vi "s.vi"() -> ()   [LabVIEW 2013] (continued)
          n587 = local read "String"() -> (w1170:string)
          n588 = Equal?(x=w1170, y=w1175) -> (x = y?=w1172:bool)
          n589 = case shown="False" w1172 {
            tunnel: w1171 -> [w1180 _]
            tunnel: [w1179 w1208] -> w1169
            tunnel: w1168 -> [w1179 _]
            frame False {
              n590 = case shown="True" w1179 {
                tunnel: w1180 -> [_ w1185]
                frame False {
                }
                frame True {
                  n591 = case shown="1" "flag 8" {
                    tunnel: [w1206 w1207] -> w1189
                    tunnel: [w1206 w1207] -> w1193
                    frame 0, Default {
                      w1206 = "Admin"
                    }
                    frame 1 {
                      w1207 = "User"
                    }
                  }
                  n592 = Concatenate Strings("String", "-" ("string"), "String", ":" ("string"), w1189) -> (w1197:string)
                  n593 = local read "Numeric"() -> (w1196:dbl)
                  n594 = Open/Create/Replace File(file path (use dialog)=path "C:/Users/kiat/Desktop/password.txt" ("file (use dialog)")) -> (refnum out=w1183:refnum<file>)  [unwired: 5 in, 2 out]
                  n595 = local read "Table Control"() -> (w1194:string[][])
                  n596 = Build Array("String", "String", w1193) -> (w1190:string[])
                  n597 = case shown="0, Default" w1196 {
                    tunnel: [w1199 w1205] -> w1182
                    tunnel: w1185 -> [w1201 w1204]
                    tunnel: w1197 -> [w1200 w1202]
                    frame 0, Default {
                      n598 = Concatenate Strings(w1201, w1200) -> (w1199:string)
                      n599 = local write "Numeric"(0.0) -> ()
                    }
                    frame 1 {
                      n600 = Concatenate Strings(w1204, "\n", w1202) -> (w1205:string)
                    }
                  }
                  n601 = Write to Text File(file (use dialog)=w1183, text=w1182) -> (refnum out=w1184:refnum<file>)  [unwired: 2 in, 2 out]
                  n602 = Insert Into Array(array=w1194, new element=w1190) -> (w1195:string[][])  [unwired: 2 in]
                  n603 = local write "Table Control"(w1195) -> ()
                  n604 = Close File(refnum=w1184) -> ()  [unwired: 1 in, 2 out]
                }
              }
            }
            frame True {
              n605 = call "Display Message to User2"("Message"="Please choose another name") -> ("OK"=w1208:bool)  [unwired: 9 in, 1 out]
            }
          }
        }
        n606 = Close File(refnum=w1167) -> ()  [unwired: 1 in, 2 out]
      }
      event "edit": Value Change {
        n607 = event-data() -> ()  [unwired: 1 in, 6 out]
        n608 = property on="Table Control" class="Tbl (strict)"() -> ("Value"=w1433:string[][])  [unwired: 2 in, 2 out]
        n609 = local read "String"() -> (w1441:string)
        n610 = Read from Text File(file (use dialog)=w1440) -> (refnum out=w1454:refnum<file>, text=w1436:string, error out=w1460:errorcluster)  [unwired: 3 in, 1 out]
        n611 = Decimal String To Number(string=w1441) -> (number=w1434:i32)  [unwired: 2 in, 1 out]
        n612 = local read "Table Control"() -> (w1447:string[][])
        n613 = Array Size(array=w1433) -> (size(s)=w1443:i32[])
        n614 = local read "String"() -> (w1444:string)
        n615 = Add(x=1, y=w1434) -> (x+y=w1435:i32)
        n616 = Close File(refnum=w1454, error in=w1460) -> (path=w1451:path, error out=w1450:errorcluster)
        n617 = Index Array(array=w1443) -> (element=w1442:i32)  [unwired: 1 in]
        n618 = Decimal String To Number(string=w1444) -> (number=w1438:i32)  [unwired: 2 in, 1 out]
        n619 = Greater Or Equal?(x=w1435, y=w1442) -> (x >= y?=w1432:bool)
        n620 = case shown="True" w1432 {
          frame False {
          }
          frame True {
            n621 = local write "Table Control"(string[][] [] ("Table Control")) -> ()
            n622 = Read from Text File(file (use dialog)=path "C:/Users/kiat/Desktop/password.txt") -> (text=w1463:string)  [unwired: 3 in, 3 out]
            n623 = while {
              border: w1463 -> [_]
              stop <- w1473 stop-if-true
              n624 = feedback #2() -> (w1477:string)
              n625 = xnode "Match Regular Expression"("input string"=w1477, "regular expression"="\n") -> ("before match"=w1476:string, "after match"=w1475:string)  [unwired: 4 in, 3 out]
              n626 = feedback-in #2(w1475) -> ()
              n627 = xnode "Match Regular Expression"("input string"=w1476, "regular expression"="-") -> ("before match"=w1472:string, "after match"=w1471:string)  [unwired: 4 in, 3 out]
              n628 = Equal?(x=w1475, y="") -> (x = y?=w1473:bool)
              n629 = xnode "Match Regular Expression"("input string"=w1471, "regular expression"=":") -> ("before match"=w1468:string, "after match"=w1469:string)  [unwired: 4 in, 3 out]
              n630 = local read "Table Control"() -> (w1465:string[][])
              n631 = Build Array(w1472, w1468, w1469) -> (w1467:string[])
              n632 = Insert Into Array(array=w1465, new element=w1467) -> (w1466:string[][])  [unwired: 2 in]
              n633 = local write "Table Control"(w1466) -> ()
            }
          }
        }
        n634 = Index Array(array=w1447, index (row)=w1438, index (col)=0 ("index")) -> (element=w1449:string)
        n635 = local read "String"() -> (w1445:string)
        n636 = local read "Table Control"() -> (w1446:string[][])
        n637 = Open/Create/Replace File(file path (use dialog)=w1451, error in=w1450, operation (0:open)=T2."replace") -> (refnum out=w1458:refnum<file>, error out=w1457:errorcluster)  [unwired: 3 in, 1 out]
        n638 = Decimal String To Number(string=w1445) -> (number=w1439:i32)  [unwired: 2 in, 1 out]
        n639 = Index Array(array=w1446, index (row)=w1439, index (col)=1 ("index")) -> (element=w1455:string)
        n640 = while {
          tunnel: w1449 -> [w1836]
          tunnel: w1455 -> [w1835]
          border: "" -> [_]
          tunnel: [w1831] -> w1453
          border: w1436 -> [_]
          stop <- w1840 stop-if-true
          n641 = feedback #3() -> (w1838:string)
          n642 = xnode "Match Regular Expression"("input string"=w1838, "regular expression"="\n") -> ("before match"=w1834:string, "after match"=w1839:string)  [unwired: 4 in, 3 out]
          n643 = feedback-in #3(w1839) -> ()
          n644 = Empty String/Path?(string/path=w1839) -> (empty?=w1840:bool)
          n645 = xnode "Match Regular Expression"("input string"=w1834, "regular expression"="-") -> ("before match"=w1828:string, "after match"=w1830:string)  [unwired: 4 in, 3 out]
          n646 = xnode "Match Regular Expression"("input string"=w1830, "regular expression"=":") -> ("before match"=w1827:string)  [unwired: 4 in, 4 out]
          n647 = local read "flag 8"() -> (w1823:u16)
          n648 = case shown="1" w1823 {
            tunnel: ["Admin" "User"] -> w1822
            frame 0, Default {
            }
            frame 1 {
            }
          }
          n649 = Equal?(x=w1836, y=w1828) -> (x = y?=w1826:bool)
          n650 = Equal?(x=w1835, y=w1827) -> (x = y?=w1825:bool)
          n651 = And(x=w1826, y=w1825) -> (x .and. y?=w1824:bool)
          n652 = case shown="True" w1824 {
            tunnel: w1834 -> [w1956 w1965]
            tunnel: [w1955 w1964] -> w1833
            tunnel: w1822 -> [_ w1958]
            frame False {
              n653 = Concatenate Strings(w1956, "\n") -> (w1955:string)
            }
            frame True {
              n654 = local read "String"() -> (w1963:string)
              n655 = local read "String"() -> (w1961:string)
              n656 = Concatenate Strings(w1963, "-" ("string"), w1961, ":" ("string"), w1958) -> (w1959:string)
              n657 = Search and Replace String(input string=w1965, search string=w1965, replace string=w1959) -> (result string=w1964:string)  [unwired: 5 in, 3 out]
            }
          }
          n658 = feedback #4() -> (w1832:string)
          n659 = Concatenate Strings(w1832, w1833) -> (w1831:string)
          n660 = feedback-in #4(w1831) -> ()
        }
        n661 = Write to Text File(file (use dialog)=w1458, text=w1453, error in=w1457) -> (refnum out=w1452:refnum<file>)  [unwired: 1 in, 2 out]
        n662 = Close File(refnum=w1452) -> ()  [unwired: 1 in, 2 out]
      }
      event "delete": Value Change {
        n663 = event-data() -> ()  [unwired: 1 in, 6 out]
        n664 = property on="Table Control" class="Tbl (strict)"() -> ("Value"=w2192:string[][])  [unwired: 2 in, 2 out]
        n665 = Read from Text File(file (use dialog)=w2196) -> (refnum out=w2203:refnum<file>, text=w2208:string, error out=w2212:errorcluster)  [unwired: 3 in, 1 out]
        n666 = local read "String"() -> (w2198:string)
        n667 = Decimal String To Number(string=w2198) -> (number=w2197:i32)  [unwired: 2 in, 1 out]
        n668 = Array Size(array=w2192) -> (size(s)=w2201:i32[])
        n669 = local read "String"() -> (w2213:string)
        n670 = Index Array(array=w2201) -> (element=w2200:i32)  [unwired: 1 in]
        n671 = local read "Table Control"() -> (w2194:string[][])
        n672 = Close File(refnum=w2203, error in=w2212) -> (path=w2191:path, error out=w2190:errorcluster)
        n673 = Greater Or Equal?(x=w2197, y=w2200) -> (x >= y?=w2199:bool)
        n674 = Decimal String To Number(string=w2213) -> (number=w2215:i32)  [unwired: 2 in, 1 out]
        n675 = Index Array(array=w2194, index (row)=w2215, index (col)=0 ("index")) -> (element=w2189:string)
        n676 = case shown="False" w2199 {
          tunnel: w2197 -> [w2218 _]
          tunnel: w2192 -> [w2217 _]
          frame False {
            n677 = Delete From Array(array=w2217, length=1, index (row)=w2218) -> (array with subset deleted=w2216:string[][])  [unwired: 1 in, 1 out]
            n678 = property on="Table Control" class="Tbl (strict)"("Value"=w2216) -> ()  [unwired: 2 in, 2 out]
          }
          frame True {
          }
        }
        n679 = local read "String"() -> (w2207:string)
        n680 = local read "Table Control"() -> (w2193:string[][])
        n681 = Open/Create/Replace File(file path (use dialog)=w2191, error in=w2190, operation (0:open)=T2."replace") -> (refnum out=w2210:refnum<file>, error out=w2209:errorcluster)  [unwired: 3 in, 1 out]
        n682 = Decimal String To Number(string=w2207) -> (number=w2205:i32)  [unwired: 2 in, 1 out]
        n683 = Index Array(array=w2193, index (row)=w2205, index (col)=1 ("index")) -> (element=w2204:string)
        n684 = while {
          tunnel: w2208 -> [w2236]
          tunnel: w2189 -> [w2233]
          tunnel: w2204 -> [w2232]
          border: "" -> [_]
          tunnel: [w2225] -> w2202
          stop <- w2239 stop-if-true
          n685 = Wait Until Next ms Multiple(millisecond multiple=u32 2000) -> ()  [unwired: 1 out]
          n686 = feedback #5(w2236) -> (w2237:string)
          n687 = xnode "Match Regular Expression"("input string"=w2237, "regular expression"="\n") -> ("before match"=w2228:string, "after match"=w2238:string)  [unwired: 4 in, 3 out]
          n688 = feedback-in #5(w2238) -> ()
          n689 = Empty String/Path?(string/path=w2238) -> (empty?=w2239:bool)
          n690 = xnode "Match Regular Expression"("input string"=w2228, "regular expression"="-") -> ("before match"=w2234:string, "after match"=w2223:string)  [unwired: 4 in, 3 out]
          n691 = xnode "Match Regular Expression"("input string"=w2223, "regular expression"=":") -> ("before match"=w2221:string)  [unwired: 4 in, 4 out]
          n692 = Equal?(x=w2233, y=w2234) -> (x = y?=w2230:bool)
          n693 = Equal?(x=w2232, y=w2221) -> (x = y?=w2231:bool)
          n694 = And(x=w2230, y=w2231) -> (x .and. y?=w2229:bool)
          n695 = case shown="False" w2229 {
            tunnel: w2228 -> [w2353 w2357]
            tunnel: [w2352 w2355] -> w2227
            frame False {
              n696 = Concatenate Strings(w2353, "\n") -> (w2352:string)
            }
            frame True {
              n697 = Search and Replace String(input string=w2357, search string=w2357, replace string="" ("replace string (\"\")")) -> (result string=w2355:string)  [unwired: 5 in, 3 out]
            }
          }
          n698 = local write "Numeric"(0.0 ("Numeric")) -> ()
          n699 = feedback #6() -> (w2226:string)
          n700 = Concatenate Strings(w2226, w2227) -> (w2225:string)
          n701 = feedback-in #6(w2225) -> ()
        }
        n702 = Write to Text File(file (use dialog)=w2210, text=w2202, error in=w2209) -> (refnum out=w2195:refnum<file>)  [unwired: 1 in, 2 out]
        n703 = Close File(refnum=w2195) -> ()  [unwired: 1 in, 2 out]
      }
      event Value Change {
        n704 = event-data() -> ()  [unwired: 1 in, 6 out]
        n705 = property class="IWMPPlayer4"(reference=w2593) -> ("settings"=w2594:refnum<k7>)  [unwired: 1 in, 2 out]
        n706 = Type Cast(x=8.0) -> (*(type *) &x=w2586:string)  [unwired: 1 in]
        n707 = TCP Write(connection ID=w2585, data in=w2586, error in (no error)=w2584) -> (connection ID out=w2588:refnum<k5>, error out=w2589:errorcluster)  [unwired: 1 in, 1 out]
        n708 = Bundle("?", 2.0) -> (w2590:cluster{dbl, dbl})  [unwired: 1 in]
        n709 = Type Cast(x=w2590) -> (*(type *) &x=w2591:string)  [unwired: 1 in]
        n710 = TCP Write(connection ID=w2588, data in=w2591, error in (no error)=w2589) -> (connection ID out=w2583:refnum<k5>, error out=w2582:errorcluster)  [unwired: 1 in, 1 out]
        n711 = property class="IWMPSettings"(reference=w2594, "volume"="?") -> (reference out=w2592:refnum<k7>)  [unwired: 1 in, 1 out]
        n712 = Close Reference(reference=w2592) -> ()  [unwired: 1 in, 1 out]
      }
      event Value Change {
        n713 = event-data() -> ()  [unwired: 1 in, 6 out]
        n714 = property on="Tab Control" class="TabCtl (strict)"("Visible"=FALSE) -> ()  [unwired: 2 in, 2 out]
        n715 = property on="Tab Control 2" class="TabCtl (strict)"("Visible"=FALSE) -> ()  [unwired: 2 in, 2 out]
        n716 = property on="Tab Control 3" class="TabCtl (strict)"("Visible"=FALSE) -> ()  [unwired: 2 in, 2 out]
        n717 = property on="Tab Control 4" class="TabCtl (strict)"("Visible"=FALSE) -> ()  [unwired: 2 in, 2 out]
        n718 = property on="Tab Control 5" class="TabCtl (strict)"("Visible"=FALSE) -> ()  [unwired: 2 in, 2 out]
        n719 = property on="Tab Control 11" class="TabCtl (strict)"("Visible"=FALSE) -> ()  [unwired: 2 in, 2 out]
        n720 = property on="Tab Control 6" class="TabCtl (strict)"("Visible"=FALSE) -> ()  [unwired: 2 in, 2 out]
        n721 = property on="Tab Control 10" class="TabCtl (strict)"("Visible"=FALSE) -> ()  [unwired: 2 in, 2 out]
        n722 = property on="Tab Control 13" class="TabCtl (strict)"("Visible"=FALSE) -> ()  [unwired: 2 in, 2 out]
        n723 = property on="Tab Control 7" class="TabCtl (strict)"("Visible"=FALSE) -> ()  [unwired: 2 in, 2 out]
        n724 = property on="Tab Control 12" class="TabCtl (strict)"("Visible"=FALSE) -> ()  [unwired: 2 in, 2 out]
        n725 = property on="Tab Control 8" class="TabCtl (strict)"("Visible"=FALSE) -> ()  [unwired: 2 in, 2 out]
        n726 = property on="Tab Control 9" class="TabCtl (strict)"("Visible"=FALSE) -> ()  [unwired: 2 in, 2 out]
        n727 = property on="Tab Control 25" class="TabCtl (strict)"("Visible"=TRUE) -> ()  [unwired: 2 in, 2 out]
        n728 = property on="Tab Control 15" class="TabCtl (strict)"("Visible"=FALSE) -> ()  [unwired: 2 in, 2 out]
        n729 = property on="Tab Control 24" class="TabCtl (strict)"("Visible"=FALSE) -> ()  [unwired: 2 in, 2 out]
        n730 = property on="Tab Control 21" class="TabCtl (strict)"("Visible"=FALSE) -> ()  [unwired: 2 in, 2 out]
        n731 = property on="Tab Control 16" class="TabCtl (strict)"("Visible"=FALSE) -> ()  [unwired: 2 in, 2 out]
        n732 = property on="Tab Control 17" class="TabCtl (strict)"("Visible"=FALSE) -> ()  [unwired: 2 in, 2 out]
        n733 = property on="Tab Control 22" class="TabCtl (strict)"("Visible"=FALSE) -> ()  [unwired: 2 in, 2 out]
        n734 = property on="Tab Control 23" class="TabCtl (strict)"("Visible"=FALSE) -> ()  [unwired: 2 in, 2 out]
        n735 = property on="Tab Control 18" class="TabCtl (strict)"("Visible"=FALSE) -> ()  [unwired: 2 in, 2 out]
        n736 = property on="Tab Control 19" class="TabCtl (strict)"("Visible"=FALSE) -> ()  [unwired: 2 in, 2 out]
        n737 = property on="Tab Control 14" class="TabCtl (strict)"("Visible"=FALSE) -> ()  [unwired: 2 in, 2 out]
      }
      event "stop": Value Change {
        n738 = event-data() -> ()  [unwired: 1 in, 6 out]
        n739 = Type Cast(x=7.0) -> (*(type *) &x=w2624:string)  [unwired: 1 in]
        n740 = TCP Write(connection ID=w2622, data in=w2624, error in (no error)=w2621) -> (connection ID out=w2626:refnum<k5>, error out=w2627:errorcluster)  [unwired: 1 in, 1 out]
        n741 = Automation Open(Automation Refnum=w2631) -> (Automation Refnum=w2632:refnum<k7>)  [unwired: 3 in, 1 out]
        n742 = property class="IWMPPlayer4"(reference=w2632) -> ("controls"=w2633:refnum<k7>)  [unwired: 1 in, 2 out]
        n743 = invoke class="IWMPControls" method="stop"(reference=w2633) -> (reference out=w2630:refnum<k7>)  [unwired: 2 in, 2 out]
        n744 = Bundle(4.0) -> (w2628:cluster{dbl})  [unwired: 1 in]
        n745 = Type Cast(x=w2628) -> (*(type *) &x=w2629:string)  [unwired: 1 in]
        n746 = Close Reference(reference=w2630) -> ()  [unwired: 1 in, 1 out]
        n747 = TCP Write(connection ID=w2626, data in=w2629, error in (no error)=w2627) -> (connection ID out=w2620:refnum<k5>, error out=w2619:errorcluster)  [unwired: 1 in, 1 out]
      }
      event Value Change {
        # "Air conditional - Master room (set temperature)"
        n748 = event-data() -> ()  [unwired: 1 in, 6 out]
        n749 = Decimal String To Number(string="String") -> (number=w2640:i32)  [unwired: 2 in, 1 out]
        n750 = Type Cast(x=6.0) -> (*(type *) &x=w2641:string)  [unwired: 1 in]
        n751 = TCP Write(connection ID=w2636, data in=w2641, error in (no error)=w2637) -> (connection ID out=w2643:refnum<k5>, error out=w2644:errorcluster)  [unwired: 1 in, 1 out]
        n752 = Bundle("?", w2640, 2.0) -> (w2645:cluster{bool, i32, dbl})  [unwired: 1 in]
        n753 = Type Cast(x=w2645) -> (*(type *) &x=w2647:string)  [unwired: 1 in]
        n754 = TCP Write(connection ID=w2643, data in=w2647, error in (no error)=w2644) -> (connection ID out=w2635:refnum<k5>, error out=w2634:errorcluster)  [unwired: 1 in, 1 out]
      }
      event Value Change {
        # "Air conditional - Bed room (set temperature)"
        n755 = event-data() -> ()  [unwired: 1 in, 6 out]
        n756 = Decimal String To Number(string="String") -> (number=w2654:i32)  [unwired: 2 in, 1 out]
        n757 = Type Cast(x=6.0) -> (*(type *) &x=w2655:string)  [unwired: 1 in]
        n758 = TCP Write(connection ID=w2650, data in=w2655, error in (no error)=w2651) -> (connection ID out=w2657:refnum<k5>, error out=w2658:errorcluster)  [unwired: 1 in, 1 out]
        n759 = Bundle("?", w2654, 3.0) -> (w2659:cluster{bool, i32, dbl})  [unwired: 1 in]
        n760 = Type Cast(x=w2659) -> (*(type *) &x=w2661:string)  [unwired: 1 in]
        n761 = TCP Write(connection ID=w2657, data in=w2661, error in (no error)=w2658) -> (connection ID out=w2653:refnum<k5>, error out=w2652:errorcluster)  [unwired: 1 in, 1 out]
      }
      event Value Change {
        n762 = event-data() -> ()  [unwired: 1 in, 6 out]
        n763 = property on="Tab Control 6" class="TabCtl (strict)"("Visible"=FALSE) -> ()  [unwired: 2 in, 2 out]
        n764 = property on="Tab Control 21" class="TabCtl (strict)"("Visible"=FALSE) -> ()  [unwired: 2 in, 2 out]
        n765 = property on="Tab Control 10" class="TabCtl (strict)"("Visible"=FALSE) -> ()  [unwired: 2 in, 2 out]
        n766 = property on="Tab Control 8" class="TabCtl (strict)"("Visible"=FALSE) -> ()  [unwired: 2 in, 2 out]
        n767 = property on="Tab Control 9" class="TabCtl (strict)"("Visible"=FALSE) -> ()  [unwired: 2 in, 2 out]
        n768 = property on="Tab Control 5" class="TabCtl (strict)"("Visible"=FALSE) -> ()  [unwired: 2 in, 2 out]
        n769 = property on="Tab Control 12" class="TabCtl (strict)"("Visible"=FALSE) -> ()  [unwired: 2 in, 2 out]
        n770 = property on="Tab Control 7" class="TabCtl (strict)"("Visible"=FALSE) -> ()  [unwired: 2 in, 2 out]
        n771 = property on="Tab Control 22" class="TabCtl (strict)"("Visible"=FALSE) -> ()  [unwired: 2 in, 2 out]
        n772 = property on="Tab Control 11" class="TabCtl (strict)"("Visible"=FALSE) -> ()  [unwired: 2 in, 2 out]
        n773 = property on="Tab Control 4" class="TabCtl (strict)"("Visible"=FALSE) -> ()  [unwired: 2 in, 2 out]
        n774 = property on="Tab Control 3" class="TabCtl (strict)"("Visible"=FALSE) -> ()  [unwired: 2 in, 2 out]
        n775 = property on="Tab Control" class="TabCtl (strict)"("Visible"=FALSE) -> ()  [unwired: 2 in, 2 out]
        n776 = property on="Tab Control 2" class="TabCtl (strict)"("Visible"=FALSE) -> ()  [unwired: 2 in, 2 out]
        n777 = property on="Tab Control 19" class="TabCtl (strict)"("Visible"=FALSE) -> ()  [unwired: 2 in, 2 out]
        n778 = property on="Tab Control 14" class="TabCtl (strict)"("Visible"=FALSE) -> ()  [unwired: 2 in, 2 out]
        n779 = property on="Tab Control 16" class="TabCtl (strict)"("Visible"=FALSE) -> ()  [unwired: 2 in, 2 out]
        n780 = property on="Tab Control 13" class="TabCtl (strict)"("Visible"=FALSE) -> ()  [unwired: 2 in, 2 out]
        n781 = property on="Tab Control 15" class="TabCtl (strict)"("Visible"=TRUE) -> ()  [unwired: 2 in, 2 out]
        n782 = property on="Tab Control 24" class="TabCtl (strict)"("Visible"=FALSE) -> ()  [unwired: 2 in, 2 out]
        n783 = property on="Tab Control 18" class="TabCtl (strict)"("Visible"=FALSE) -> ()  [unwired: 2 in, 2 out]
        n784 = property on="Tab Control 17" class="TabCtl (strict)"("Visible"=FALSE) -> ()  [unwired: 2 in, 2 out]
      }
      event Value Change {
        n785 = event-data() -> ()  [unwired: 1 in, 6 out]
        n786 = Type Cast(x=4.0) -> (*(type *) &x=w2689:string)  [unwired: 1 in]
        n787 = TCP Write(connection ID=w2687, data in=w2689, error in (no error)=w2684) -> (connection ID out=w2686:refnum<k5>, error out=w2685:errorcluster)  [unwired: 1 in, 1 out]
        n788 = Bundle("?", 12.0) -> (w2694:cluster{bool, dbl})  [unwired: 1 in]
        n789 = Type Cast(x=w2694) -> (*(type *) &x=w2695:string)  [unwired: 1 in]
        n790 = TCP Write(connection ID=w2686, data in=w2695, error in (no error)=w2685) -> (connection ID out=w2692:refnum<k5>, error out=w2691:errorcluster)  [unwired: 1 in, 1 out]
      }
      event "OK Button 31": Value Change {
        n791 = event-data() -> ()  [unwired: 1 in, 6 out]
        n792 = Type Cast(x=4.0) -> (*(type *) &x=w2701:string)  [unwired: 1 in]
        n793 = TCP Write(connection ID=w2697, data in=w2701, error in (no error)=w2696) -> (connection ID out=w2698:refnum<k5>, error out=w2699:errorcluster)  [unwired: 1 in, 1 out]
        n794 = Bundle("OK Button 31"="OK Button 31", 13.0) -> (w2706:cluster{"OK Button 31":bool, dbl})  [unwired: 1 in]
        n795 = Type Cast(x=w2706) -> (*(type *) &x=w2707:string)  [unwired: 1 in]
        n796 = TCP Write(connection ID=w2698, data in=w2707, error in (no error)=w2699) -> (connection ID out=w2705:refnum<k5>, error out=w2704:errorcluster)  [unwired: 1 in, 1 out]
      }
      event "OK Button 32": Value Change {
        n797 = event-data() -> ()  [unwired: 1 in, 6 out]
        n798 = Type Cast(x=4.0) -> (*(type *) &x=w2716:string)  [unwired: 1 in]
        n799 = TCP Write(connection ID=w2709, data in=w2716, error in (no error)=w2710) -> (connection ID out=w2713:refnum<k5>, error out=w2714:errorcluster)  [unwired: 1 in, 1 out]
        n800 = Bundle("OK Button 32"="OK Button 32", 14.0) -> (w2718:cluster{"OK Button 32":bool, dbl})  [unwired: 1 in]
        n801 = Type Cast(x=w2718) -> (*(type *) &x=w2719:string)  [unwired: 1 in]
        n802 = TCP Write(connection ID=w2713, data in=w2719, error in (no error)=w2714) -> (connection ID out=w2712:refnum<k5>, error out=w2711:errorcluster)  [unwired: 1 in, 1 out]
      }
      event Value Change {
        n803 = event-data() -> ()  [unwired: 1 in, 6 out]
        n804 = Type Cast(x=4.0) -> (*(type *) &x=w2724:string)  [unwired: 1 in]
        n805 = TCP Write(connection ID=w2721, data in=w2724, error in (no error)=w2722) -> (connection ID out=w2720:refnum<k5>, error out=w2723:errorcluster)  [unwired: 1 in, 1 out]
        n806 = Bundle("?", 1.0) -> (w2730:cluster{bool, dbl})  [unwired: 1 in]
        n807 = Type Cast(x=w2730) -> (*(type *) &x=w2731:string)  [unwired: 1 in]
        n808 = TCP Write(connection ID=w2720, data in=w2731, error in (no error)=w2723) -> (connection ID out=w2728:refnum<k5>, error out=w2729:errorcluster)  [unwired: 1 in, 1 out]
      }
      event "OK Button 19": Value Change {
        n809 = event-data() -> ()  [unwired: 1 in, 6 out]
        n810 = Type Cast(x=4.0) -> (*(type *) &x=w2737:string)  [unwired: 1 in]
        n811 = TCP Write(connection ID=w2734, data in=w2737, error in (no error)=w2735) -> (connection ID out=w2733:refnum<k5>, error out=w2732:errorcluster)  [unwired: 1 in, 1 out]
        n812 = Bundle("OK Button 19"="OK Button 19", 2.0) -> (w2741:cluster{"OK Button 19":bool, dbl})  [unwired: 1 in]
        n813 = Type Cast(x=w2741) -> (*(type *) &x=w2743:string)  [unwired: 1 in]
        n814 = TCP Write(connection ID=w2733, data in=w2743, error in (no error)=w2732) -> (connection ID out=w2739:refnum<k5>, error out=w2740:errorcluster)  [unwired: 1 in, 1 out]
      }
      event "OK Button 20": Value Change {
        n815 = event-data() -> ()  [unwired: 1 in, 6 out]
        n816 = Type Cast(x=4.0) -> (*(type *) &x=w2749:string)  [unwired: 1 in]
        n817 = TCP Write(connection ID=w2746, data in=w2749, error in (no error)=w2747) -> (connection ID out=w2745:refnum<k5>, error out=w2744:errorcluster)  [unwired: 1 in, 1 out]
        n818 = Bundle("OK Button 20"="OK Button 20", 3.0) -> (w2750:cluster{"OK Button 20":bool, dbl})  [unwired: 1 in]
        n819 = Type Cast(x=w2750) -> (*(type *) &x=w2755:string)  [unwired: 1 in]
        n820 = TCP Write(connection ID=w2745, data in=w2755, error in (no error)=w2744) -> (connection ID out=w2753:refnum<k5>, error out=w2752:errorcluster)  [unwired: 1 in, 1 out]
      }
      event "OK Button 21": Value Change {
        n821 = event-data() -> ()  [unwired: 1 in, 6 out]
        n822 = Type Cast(x=4.0) -> (*(type *) &x=w2761:string)  [unwired: 1 in]
        n823 = TCP Write(connection ID=w2759, data in=w2761, error in (no error)=w2758) -> (connection ID out=w2756:refnum<k5>, error out=w2757:errorcluster)  [unwired: 1 in, 1 out]
        n824 = Bundle("OK Button 21"="OK Button 21", 4.0) -> (w2766:cluster{"OK Button 21":bool, dbl})  [unwired: 1 in]
        n825 = Type Cast(x=w2766) -> (*(type *) &x=w2767:string)  [unwired: 1 in]
        n826 = TCP Write(connection ID=w2756, data in=w2767, error in (no error)=w2757) -> (connection ID out=w2764:refnum<k5>, error out=w2763:errorcluster)  [unwired: 1 in, 1 out]
      }
      event "OK Button 22": Value Change {
        n827 = event-data() -> ()  [unwired: 1 in, 6 out]
        n828 = Type Cast(x=4.0) -> (*(type *) &x=w2773:string)  [unwired: 1 in]
        n829 = TCP Write(connection ID=w2770, data in=w2773, error in (no error)=w2769) -> (connection ID out=w2771:refnum<k5>, error out=w2768:errorcluster)  [unwired: 1 in, 1 out]
        n830 = Bundle("OK Button 22"="OK Button 22", 5.0) -> (w2778:cluster{"OK Button 22":bool, dbl})  [unwired: 1 in]
        n831 = Type Cast(x=w2778) -> (*(type *) &x=w2779:string)  [unwired: 1 in]
        n832 = TCP Write(connection ID=w2771, data in=w2779, error in (no error)=w2768) -> (connection ID out=w2776:refnum<k5>, error out=w2775:errorcluster)  [unwired: 1 in, 1 out]
      }
      event "OK Button 23": Value Change {
        n833 = event-data() -> ()  [unwired: 1 in, 6 out]
        n834 = Type Cast(x=4.0) -> (*(type *) &x=w2780:string)  [unwired: 1 in]
        n835 = TCP Write(connection ID=w2784, data in=w2780, error in (no error)=w2783) -> (connection ID out=w2781:refnum<k5>, error out=w2782:errorcluster)  [unwired: 1 in, 1 out]
        n836 = Bundle("OK Button 23"="OK Button 23", 6.0) -> (w2790:cluster{"OK Button 23":bool, dbl})  [unwired: 1 in]
        n837 = Type Cast(x=w2790) -> (*(type *) &x=w2791:string)  [unwired: 1 in]
        n838 = TCP Write(connection ID=w2781, data in=w2791, error in (no error)=w2782) -> (connection ID out=w2788:refnum<k5>, error out=w2787:errorcluster)  [unwired: 1 in, 1 out]
      }
      event "OK Button 24": Value Change {
        n839 = event-data() -> ()  [unwired: 1 in, 6 out]
        n840 = Type Cast(x=4.0) -> (*(type *) &x=w2792:string)  [unwired: 1 in]
        n841 = TCP Write(connection ID=w2797, data in=w2792, error in (no error)=w2796) -> (connection ID out=w2798:refnum<k5>, error out=w2799:errorcluster)  [unwired: 1 in, 1 out]
        n842 = Bundle("OK Button 24"="OK Button 24", 7.0) -> (w2802:cluster{"OK Button 24":bool, dbl})  [unwired: 1 in]
        n843 = Type Cast(x=w2802) -> (*(type *) &x=w2803:string)  [unwired: 1 in]
        n844 = TCP Write(connection ID=w2798, data in=w2803, error in (no error)=w2799) -> (connection ID out=w2795:refnum<k5>, error out=w2794:errorcluster)  [unwired: 1 in, 1 out]
      }
      event Value Change {
        n845 = event-data() -> ()  [unwired: 1 in, 6 out]
        n846 = Type Cast(x=4.0) -> (*(type *) &x=w2809:string)  [unwired: 1 in]
        n847 = TCP Write(connection ID=w2805, data in=w2809, error in (no error)=w2804) -> (connection ID out=w2806:refnum<k5>, error out=w2807:errorcluster)  [unwired: 1 in, 1 out]
        n848 = Bundle("?", 8.0) -> (w2814:cluster{bool, dbl})  [unwired: 1 in]
        n849 = Type Cast(x=w2814) -> (*(type *) &x=w2815:string)  [unwired: 1 in]
        n850 = TCP Write(connection ID=w2806, data in=w2815, error in (no error)=w2807) -> (connection ID out=w2811:refnum<k5>, error out=w2810:errorcluster)  [unwired: 1 in, 1 out]
      }
      event "OK Button 25": Value Change {
        n851 = event-data() -> ()  [unwired: 1 in, 6 out]
        n852 = Type Cast(x=4.0) -> (*(type *) &x=w2821:string)  [unwired: 1 in]
        n853 = TCP Write(connection ID=w2816, data in=w2821, error in (no error)=w2819) -> (connection ID out=w2817:refnum<k5>, error out=w2818:errorcluster)  [unwired: 1 in, 1 out]
        n854 = Bundle("OK Button 25"="OK Button 25", 9.0) -> (w2826:cluster{"OK Button 25":bool, dbl})  [unwired: 1 in]
        n855 = Type Cast(x=w2826) -> (*(type *) &x=w2827:string)  [unwired: 1 in]
        n856 = TCP Write(connection ID=w2817, data in=w2827, error in (no error)=w2818) -> (connection ID out=w2824:refnum<k5>, error out=w2823:errorcluster)  [unwired: 1 in, 1 out]
      }
      event "OK Button 26": Value Change {
        n857 = event-data() -> ()  [unwired: 1 in, 6 out]
        n858 = Type Cast(x=4.0) -> (*(type *) &x=w2833:string)  [unwired: 1 in]
        n859 = TCP Write(connection ID=w2831, data in=w2833, error in (no error)=w2830) -> (connection ID out=w2829:refnum<k5>, error out=w2828:errorcluster)  [unwired: 1 in, 1 out]
        n860 = Bundle("OK Button 26"="OK Button 26", 10.0) -> (w2838:cluster{"OK Button 26":bool, dbl})  [unwired: 1 in]
        n861 = Type Cast(x=w2838) -> (*(type *) &x=w2839:string)  [unwired: 1 in]
        n862 = TCP Write(connection ID=w2829, data in=w2839, error in (no error)=w2828) -> (connection ID out=w2836:refnum<k5>, error out=w2835:errorcluster)  [unwired: 1 in, 1 out]
      }
      event "OK Button 27": Value Change {
        n863 = event-data() -> ()  [unwired: 1 in, 6 out]
        n864 = Type Cast(x=4.0) -> (*(type *) &x=w2845:string)  [unwired: 1 in]
        n865 = TCP Write(connection ID=w2843, data in=w2845, error in (no error)=w2840) -> (connection ID out=w2842:refnum<k5>, error out=w2841:errorcluster)  [unwired: 1 in, 1 out]
        n866 = Bundle("OK Button 27"="OK Button 27", 11.0) -> (w2850:cluster{"OK Button 27":bool, dbl})  [unwired: 1 in]
        n867 = Type Cast(x=w2850) -> (*(type *) &x=w2851:string)  [unwired: 1 in]
        n868 = TCP Write(connection ID=w2842, data in=w2851, error in (no error)=w2841) -> (connection ID out=w2848:refnum<k5>, error out=w2847:errorcluster)  [unwired: 1 in, 1 out]
      }
      event Value Change {
        (unwired) FALSE ("Visible")
        n869 = event-data() -> ()  [unwired: 1 in, 6 out]
        n870 = property on="Tab Control 8" class="TabCtl (strict)"("Visible"=FALSE) -> ()  [unwired: 2 in, 2 out]
        n871 = property on="Tab Control 6" class="TabCtl (strict)"("Visible"=FALSE) -> ()  [unwired: 2 in, 2 out]
        n872 = property on="Tab Control 9" class="TabCtl (strict)"("Visible"=FALSE) -> ()  [unwired: 2 in, 2 out]
        n873 = property on="Tab Control 19" class="TabCtl (strict)"("Visible"=FALSE) -> ()  [unwired: 2 in, 2 out]
        n874 = property on="Tab Control 22" class="TabCtl (strict)"("Visible"=FALSE) -> ()  [unwired: 2 in, 2 out]
        n875 = property on="Tab Control 12" class="TabCtl (strict)"("Visible"=FALSE) -> ()  [unwired: 2 in, 2 out]
        n876 = property on="Tab Control 5" class="TabCtl (strict)"("Visible"=TRUE) -> ()  [unwired: 2 in, 2 out]
        n877 = property on="Tab Control 4" class="TabCtl (strict)"("Visible"=FALSE) -> ()  [unwired: 2 in, 2 out]
        n878 = property on="Tab Control 3" class="TabCtl (strict)"("Visible"=FALSE) -> ()  [unwired: 2 in, 2 out]
        n879 = property on="Tab Control" class="TabCtl (strict)"("Visible"=FALSE) -> ()  [unwired: 2 in, 2 out]
        n880 = property on="Tab Control 2" class="TabCtl (strict)"("Visible"=FALSE) -> ()  [unwired: 2 in, 2 out]
        n881 = property on="Tab Control 21" class="TabCtl (strict)"("Visible"=FALSE) -> ()  [unwired: 2 in, 2 out]
        n882 = property on="Tab Control 10" class="TabCtl (strict)"("Visible"=FALSE) -> ()  [unwired: 2 in, 2 out]
        n883 = property on="Tab Control 7" class="TabCtl (strict)"("Visible"=FALSE) -> ()  [unwired: 2 in, 2 out]
        n884 = property on="Tab Control 11" class="TabCtl (strict)"("Visible"=FALSE) -> ()  [unwired: 2 in, 2 out]
        n885 = property on="Tab Control 16" class="TabCtl (strict)"("Visible"=FALSE) -> ()  [unwired: 2 in, 2 out]
        n886 = property on="Tab Control 14" class="TabCtl (strict)"("Visible"=FALSE) -> ()  [unwired: 2 in, 2 out]
        n887 = property on="Tab Control 13" class="TabCtl (strict)"("Visible"=FALSE) -> ()  [unwired: 2 in, 2 out]
        n888 = property on="Tab Control 15" class="TabCtl (strict)"("Visible"=FALSE) -> ()  [unwired: 2 in, 2 out]
        n889 = property on="Tab Control 18" class="TabCtl (strict)"("Visible"=FALSE) -> ()  [unwired: 2 in, 2 out]
        n890 = property on="Tab Control 17" class="TabCtl (strict)"("Visible"=FALSE) -> ()  [unwired: 2 in, 2 out]
        n891 = property on="Tab Control 24" class="TabCtl (strict)"("Visible"=FALSE) -> ()  [unwired: 2 in, 2 out]
      }
      event Value Change {
        n892 = event-data() -> ()  [unwired: 1 in, 6 out]
        n893 = Type Cast(x=0.0) -> ()  [unwired: 1 in, 1 out]
        n894 = TCP Write(connection ID=w2874, error in (no error)=w2875) -> (connection ID out=w2877:refnum<k5>, error out=w2876:errorcluster)  [unwired: 2 in, 1 out]
        n895 = Bundle("?", 3.0) -> (w2883:cluster{bool, dbl})  [unwired: 1 in]
        n896 = Type Cast(x=w2883) -> (*(type *) &x=w2884:string)  [unwired: 1 in]
        n897 = TCP Write(connection ID=w2877, data in=w2884, error in (no error)=w2876) -> (connection ID out=w2880:refnum<k5>, error out=w2879:errorcluster)  [unwired: 1 in, 1 out]
      }
      event "OK Button 11": Value Change {
        n898 = event-data() -> ()  [unwired: 1 in, 6 out]
        n899 = Type Cast(x=0.0) -> (*(type *) &x=w2890:string)  [unwired: 1 in]
        n900 = TCP Write(connection ID=w2887, data in=w2890, error in (no error)=w2888) -> (connection ID out=w2886:refnum<k5>, error out=w2885:errorcluster)  [unwired: 1 in, 1 out]
        n901 = Bundle("OK Button 11"="OK Button 11", 4.0) -> (w2895:cluster{"OK Button 11":bool, dbl})  [unwired: 1 in]
        n902 = Type Cast(x=w2895) -> (*(type *) &x=w2896:string)  [unwired: 1 in]
        n903 = TCP Write(connection ID=w2886, data in=w2896, error in (no error)=w2885) -> (connection ID out=w2892:refnum<k5>, error out=w2891:errorcluster)  [unwired: 1 in, 1 out]
      }
      event "OK Button 12": Value Change {
        n904 = event-data() -> ()  [unwired: 1 in, 6 out]
        n905 = Type Cast(x=0.0) -> (*(type *) &x=w2902:string)  [unwired: 1 in]
        n906 = TCP Write(connection ID=w2900, data in=w2902, error in (no error)=w2897) -> (connection ID out=w2899:refnum<k5>, error out=w2898:errorcluster)  [unwired: 1 in, 1 out]
        n907 = Bundle("OK Button 12"="OK Button 12", 8.0) -> (w2907:cluster{"OK Button 12":bool, dbl})  [unwired: 1 in]
        n908 = Type Cast(x=w2907) -> (*(type *) &x=w2908:string)  [unwired: 1 in]
        n909 = TCP Write(connection ID=w2899, data in=w2908, error in (no error)=w2898) -> (connection ID out=w2904:refnum<k5>, error out=w2905:errorcluster)  [unwired: 1 in, 1 out]
      }
      event "OK Button 13": Value Change {
        n910 = event-data() -> ()  [unwired: 1 in, 6 out]
        n911 = Type Cast(x=0.0) -> (*(type *) &x=w2914:string)  [unwired: 1 in]
        n912 = TCP Write(connection ID=w2912, data in=w2914, error in (no error)=w2909) -> (connection ID out=w2911:refnum<k5>, error out=w2910:errorcluster)  [unwired: 1 in, 1 out]
        n913 = Bundle("OK Button 13"="OK Button 13", 9.0) -> (w2919:cluster{"OK Button 13":bool, dbl})  [unwired: 1 in]
        n914 = Type Cast(x=w2919) -> (*(type *) &x=w2920:string)  [unwired: 1 in]
        n915 = TCP Write(connection ID=w2911, data in=w2920, error in (no error)=w2910) -> (connection ID out=w2916:refnum<k5>, error out=w2917:errorcluster)  [unwired: 1 in, 1 out]
      }
      event "OK Button 14": Value Change {
        n916 = event-data() -> ()  [unwired: 1 in, 6 out]
        n917 = Type Cast(x=0.0) -> ()  [unwired: 1 in, 1 out]
        n918 = TCP Write(connection ID=w2922, error in (no error)=w2921) -> (connection ID out=w2923:refnum<k5>, error out=w2924:errorcluster)  [unwired: 2 in, 1 out]
        n919 = Bundle("OK Button 14"="OK Button 14", 19.0) -> (w2930:cluster{"OK Button 14":bool, dbl})  [unwired: 1 in]
        n920 = Type Cast(x=w2930) -> (*(type *) &x=w2931:string)  [unwired: 1 in]
        n921 = TCP Write(connection ID=w2923, data in=w2931, error in (no error)=w2924) -> (connection ID out=w2928:refnum<k5>, error out=w2929:errorcluster)  [unwired: 1 in, 1 out]
      }
      event Value Change {
        n922 = event-data() -> ()  [unwired: 1 in, 6 out]
        n923 = Type Cast(x=0.0) -> (*(type *) &x=w2937:string)  [unwired: 1 in]
        n924 = TCP Write(connection ID=w2933, data in=w2937, error in (no error)=w2932) -> (connection ID out=w2934:refnum<k5>, error out=w2935:errorcluster)  [unwired: 1 in, 1 out]
        n925 = Bundle("?", 1.0) -> (w2940:cluster{bool, dbl})  [unwired: 1 in]
        n926 = Type Cast(x=w2940) -> (*(type *) &x=w2941:string)  [unwired: 1 in]
        n927 = TCP Write(connection ID=w2934, data in=w2941, error in (no error)=w2935) -> (connection ID out=w2943:refnum<k5>, error out=w2942:errorcluster)  [unwired: 1 in, 1 out]
      }
      event "OK Button 5": Value Change {
        n928 = event-data() -> ()  [unwired: 1 in, 6 out]
        n929 = Type Cast(x=0.0) -> (*(type *) &x=w2944:string)  [unwired: 1 in]
        n930 = TCP Write(connection ID=w2947, data in=w2944, error in (no error)=w2948) -> (connection ID out=w2946:refnum<k5>, error out=w2945:errorcluster)  [unwired: 1 in, 1 out]
        n931 = Bundle("OK Button 5"="OK Button 5", 2.0) -> (w2954:cluster{"OK Button 5":bool, dbl})  [unwired: 1 in]
        n932 = Type Cast(x=w2954) -> (*(type *) &x=w2955:string)  [unwired: 1 in]
        n933 = TCP Write(connection ID=w2946, data in=w2955, error in (no error)=w2945) -> (connection ID out=w2951:refnum<k5>, error out=w2950:errorcluster)  [unwired: 1 in, 1 out]
      }
      event Value Change {
        n934 = event-data() -> ()  [unwired: 1 in, 6 out]
        n935 = Add(x=u16 1, y="start hour 1") -> (x+y=w2961:u16)
        n936 = To Double Precision Float(number=w2961) -> (double precision float=w2973:dbl)
        n937 = To Double Precision Float(number="start min 1") -> (double precision float=w2972:dbl)
        n938 = Type Cast(x=3.0) -> (*(type *) &x=w2979:string)  [unwired: 1 in]
        n939 = TCP Write(connection ID=w2975, data in=w2979, error in (no error)=w2974) -> (connection ID out=w2976:refnum<k5>, error out=w2980:errorcluster)  [unwired: 1 in, 1 out]
        n940 = Add(x="end hour 1", y=u16 1) -> (x+y=w2959:u16)
        n941 = To Double Precision Float(number="end min 1") -> (double precision float=w2965:dbl)
        n942 = To Double Precision Float(number=w2959) -> (double precision float=w2964:dbl)
        n943 = To Double Precision Float(number="flag") -> (double precision float=w2967:dbl)
        n944 = To Double Precision Float(number="flag 2") -> (double precision float=w2969:dbl)
        n945 = Bundle(w2973, w2972, w2964, w2965, w2967, w2969, 1, "?") -> (w2982:cluster{dbl, dbl, dbl, dbl, dbl, dbl, i32, bool})  [unwired: 1 in]
        n946 = Type Cast(x=w2982) -> (*(type *) &x=w2983:string)  [unwired: 1 in]
        n947 = TCP Write(connection ID=w2976, data in=w2983, error in (no error)=w2980) -> (connection ID out=w2977:refnum<k5>, error out=w2978:errorcluster)  [unwired: 1 in, 1 out]
      }
      event Value Change {
        n948 = event-data() -> ()  [unwired: 1 in, 6 out]
        n949 = Add(x=u16 1, y="start hour 2") -> (x+y=w2995:u16)
        n950 = To Double Precision Float(number=w2995) -> (double precision float=w3003:dbl)
        n951 = To Double Precision Float(number="start min 2") -> (double precision float=w3002:dbl)
        n952 = Add(x="end hour 2", y=u16 1) -> (x+y=w2994:u16)
        n953 = To Double Precision Float(number="end min 2") -> (double precision float=w2998:dbl)
        n954 = To Double Precision Float(number=w2994) -> (double precision float=w2997:dbl)
        n955 = Type Cast(x=3.0) -> (*(type *) &x=w3009:string)  [unwired: 1 in]
        n956 = TCP Write(connection ID=w3005, data in=w3009, error in (no error)=w3004) -> (connection ID out=w3008:refnum<k5>, error out=w3010:errorcluster)  [unwired: 1 in, 1 out]
        n957 = To Double Precision Float(number="flag 3") -> (double precision float=w3000:dbl)
        n958 = To Double Precision Float(number="flag 4") -> (double precision float=w3001:dbl)
        n959 = Bundle(w3003, w3002, w2997, w2998, w3000, w3001, 2, "?") -> (w2986:cluster{dbl, dbl, dbl, dbl, dbl, dbl, i32, bool})  [unwired: 1 in]
        n960 = Type Cast(x=w2986) -> (*(type *) &x=w2985:string)  [unwired: 1 in]
        n961 = TCP Write(connection ID=w3008, data in=w2985, error in (no error)=w3010) -> (connection ID out=w3006:refnum<k5>, error out=w3007:errorcluster)  [unwired: 1 in, 1 out]
      }
      event Value Change {
        n962 = event-data() -> ()  [unwired: 1 in, 6 out]
        n963 = Add(x=u16 1, y="start hour 3") -> (x+y=w3025:u16)
        n964 = To Double Precision Float(number=w3025) -> (double precision float=w3032:dbl)
        n965 = To Double Precision Float(number="start min 3") -> (double precision float=w3031:dbl)
        n966 = Add(x="end hour 3", y=u16 1) -> (x+y=w3024:u16)
        n967 = To Double Precision Float(number="end min 3") -> (double precision float=w3028:dbl)
        n968 = To Double Precision Float(number=w3024) -> (double precision float=w3027:dbl)
        n969 = Type Cast(x=3.0) -> (*(type *) &x=w3021:string)  [unwired: 1 in]
        n970 = TCP Write(connection ID=w3035, data in=w3021, error in (no error)=w3034) -> (connection ID out=w3038:refnum<k5>, error out=w3039:errorcluster)  [unwired: 1 in, 1 out]
        n971 = To Double Precision Float(number="flag 5") -> (double precision float=w3029:dbl)
        n972 = To Double Precision Float(number="flag 6") -> (double precision float=w3030:dbl)
        n973 = Bundle(w3032, w3031, w3027, w3028, w3029, w3030, 3, "?") -> (w3022:cluster{dbl, dbl, dbl, dbl, dbl, dbl, i32, bool})  [unwired: 1 in]
        n974 = Type Cast(x=w3022) -> (*(type *) &x=w3020:string)  [unwired: 1 in]
        n975 = TCP Write(connection ID=w3038, data in=w3020, error in (no error)=w3039) -> (connection ID out=w3036:refnum<k5>, error out=w3037:errorcluster)  [unwired: 1 in, 1 out]
      }
      event Value Change {
        # "Air conditional menu"
        n976 = event-data() -> ()  [unwired: 1 in, 6 out]
        n977 = property on="Tab Control" class="TabCtl (strict)"("Visible"=FALSE) -> ()  [unwired: 2 in, 2 out]
        n978 = property on="Tab Control 2" class="TabCtl (strict)"("Visible"=FALSE) -> ()  [unwired: 2 in, 2 out]
        n979 = property on="Tab Control 3" class="TabCtl (strict)"("Visible"=FALSE) -> ()  [unwired: 2 in, 2 out]
        n980 = property on="Tab Control 4" class="TabCtl (strict)"("Visible"=FALSE) -> ()  [unwired: 2 in, 2 out]
        n981 = property on="Tab Control 5" class="TabCtl (strict)"("Visible"=FALSE) -> ()  [unwired: 2 in, 2 out]
        n982 = property on="Tab Control 13" class="TabCtl (strict)"("Visible"=FALSE) -> ()  [unwired: 2 in, 2 out]
        n983 = property on="Tab Control 14" class="TabCtl (strict)"("Visible"=FALSE) -> ()  [unwired: 2 in, 2 out]
        n984 = property on="Tab Control 11" class="TabCtl (strict)"("Visible"=FALSE) -> ()  [unwired: 2 in, 2 out]
        n985 = property on="Tab Control 6" class="TabCtl (strict)"("Visible"=FALSE) -> ()  [unwired: 2 in, 2 out]
        n986 = property on="Tab Control 10" class="TabCtl (strict)"("Visible"=FALSE) -> ()  [unwired: 2 in, 2 out]
        n987 = property on="Tab Control 7" class="TabCtl (strict)"("Visible"=FALSE) -> ()  [unwired: 2 in, 2 out]
        n988 = property on="Tab Control 12" class="TabCtl (strict)"("Visible"=FALSE) -> ()  [unwired: 2 in, 2 out]
        n989 = property on="Tab Control 8" class="TabCtl (strict)"("Visible"=FALSE) -> ()  [unwired: 2 in, 2 out]
        n990 = property on="Tab Control 9" class="TabCtl (strict)"("Visible"=FALSE) -> ()  [unwired: 2 in, 2 out]